vi "Dresden R2R Sputter 03.02.2018 IY24.vi"() -> ()   [LabVIEW 2009] (continued)
                        n5703 = while {
                          i -> [w8756]
                          stop <- w8751 stop-if-true
                          n5704 = Greater?(x=w8756, y=100) -> (0:w8752:bool)
                          n5705 = Wait Until Next ms Multiple(millisecond multiple=u32 300) -> ()  [unwired: 1 out]
                          n5706 = local read "Parameters_auto_set"() -> (w8757:bool)
                          n5707 = case shown="False" w8757 {
                            tunnel: [TRUE FALSE] -> w8753
                            frame #0 {
                            }
                            frame #1 {
                            }
                          }
                          n5708 = Or(x=w8753, y=w8752) -> (x .or. y?=w8751:bool)
                        }
                      }
                      frame #9 {
                        n5709 = local write "Start_roll"(TRUE ("Start_roll")) -> ()
                      }
                      frame #10 {
                        n5710 = while {
                          stop <- w8762 stop-if-true
                          n5711 = local read "Actual Length"() -> (w8766:dbl)
                          n5712 = local read "Region"() -> (w8765:dbl)
                          n5713 = local read "Semi"() -> (w8763:bool)
                          n5714 = Greater Or Equal?(x=w8766, y=w8765) -> (x >= y?=w8764:bool)
                          n5715 = Or(x=w8764, y=w8763) -> (x .or. y?=w8762:bool)
                          n5716 = Wait Until Next ms Multiple(millisecond multiple=u32 300) -> ()  [unwired: 1 out]
                        }
                      }
                      frame #11 {
                        n5717 = local write "Start_full_foil"(FALSE ("Start_full_foil")) -> ()
                      }
                    }
                  }
                }
              }
              frame #1 {
                n5718 = local read "Roll_side_select 2"() -> (w8768:enum32{"Left to Right", "Right to Left"})
                n5719 = case shown="\"Right to Left\"" w8768 {
                  frame #0 {
                    n5720 = stacked-sequence {
                      frame #0 {
                        n5721 = local read "Target_length_left side"() -> (w8772:dbl)
                        n5722 = local read "Max Diameter 2"() -> (w8775:dbl)
                        n5723 = local read "Min Diameter 2"() -> (w8774:dbl)
                        n5724 = local read "Web Speed 2"() -> (w8770:dbl)
                        n5725 = local read "Web_Thickness2"() -> (w8769:dbl)
                        n5726 = local write "Initial Min Diameter"(w8774) -> ()
                        n5727 = local write "Web Speed"(w8770) -> ()
                        n5728 = local write "Max Diameter"(w8775) -> ()
                        n5729 = local write "Roll_side_select"(enum32{"Left to Right", "Right to Left"}."Left to Right" ("Roll_side_select")) -> ()
                        n5730 = local write "Region"(w8772) -> ()
                        n5731 = local write "Web Thickness"(w8769) -> ()
                        n5732 = Wait (ms)(milliseconds to wait=u32 1000) -> ()  [unwired: 1 out]
                      }
                      frame #1 {
                        n5733 = local write "Calculate 2"(TRUE ("Calculate_auto")) -> ()
                      }
                      frame #2 {
                        n5734 = local read "Tension_Value2"() -> (w8778:dbl)
                        n5735 = Wait (ms)(milliseconds to wait=u32 300) -> ()  [unwired: 1 out]
                        n5736 = local write "TC1_set_value"(w8778) -> ()
                      }
                      frame #3 {
                        w8779 = u16 1 items=["1", "2", "3", "4"] ("Target Chamber Sensor")
                        n5737 = local write "Target Chamber Sensor"(w8779) -> ()
                      }
                      frame #4 {
                        n5738 = local write "TC1_set"(TRUE ("TC1_set")) -> ()
                      }
                      frame #5 {
                        n5739 = local write "Parameters_auto_set"(TRUE ("Parameters_auto_set")) -> ()
                      }
                      frame #6 {
                        n5740 = while {
                          i -> [w8787]
                          stop <- w8782 stop-if-true
                          n5741 = Greater?(x=w8787, y=100) -> (0:w8783:bool)
                          n5742 = Wait Until Next ms Multiple(millisecond multiple=u32 300) -> ()  [unwired: 1 out]
                          n5743 = local read "Parameters_auto_set"() -> (w8788:bool)
                          n5744 = case shown="False" w8788 {
                            tunnel: [TRUE FALSE] -> w8784
                            frame #0 {
                            }
                            frame #1 {
                            }
                          }
                          n5745 = Or(x=w8784, y=w8783) -> (x .or. y?=w8782:bool)
                        }
                      }
                      frame #7 {
                        n5746 = local write "Start_roll"(TRUE ("Start_roll")) -> ()
                      }
                      frame #8 {
                        n5747 = while {
                          stop <- w8793 stop-if-true
                          n5748 = local read "Actual Length"() -> (w8797:dbl)
                          n5749 = local read "Region"() -> (w8796:dbl)
                          n5750 = local read "Semi"() -> (w8794:bool)
                          n5751 = Greater Or Equal?(x=w8797, y=w8796) -> (x >= y?=w8795:bool)
                          n5752 = Or(x=w8795, y=w8794) -> (x .or. y?=w8793:bool)
                          n5753 = Wait Until Next ms Multiple(millisecond multiple=u32 300) -> ()  [unwired: 1 out]
                        }
                      }
                      frame #9 {
                        n5754 = local write "Start_full_foil"(FALSE ("Start_full_foil")) -> ()
                      }
                    }
                  }
                  frame #1 {
                    n5755 = stacked-sequence {
                      frame #0 {
                        n5756 = local read "Target_length_right side"() -> (w8803:dbl)
                        n5757 = local read "Web_Thickness2"() -> (w8799:dbl)
                        n5758 = local read "Max Diameter 2"() -> (w8804:dbl)
                        n5759 = local read "Web Speed 2"() -> (w8800:dbl)
                        n5760 = local write "Web Speed"(w8800) -> ()
                        n5761 = local write "Max Diameter"(w8804) -> ()
                        n5762 = local write "Roll_side_select"(enum32{"Left to Right", "Right to Left"}."Right to Left" ("Roll_side_select")) -> ()
                        n5763 = local write "Web Thickness"(w8799) -> ()
                        n5764 = local write "Region"(w8803) -> ()
                        n5765 = Wait (ms)(milliseconds to wait=u32 1000) -> ()  [unwired: 1 out]
                      }
                      frame #1 {
                        n5766 = local write "Calculate 3"(TRUE ("Calculate_auto")) -> ()
                      }
                      frame #2 {
                        n5767 = local read "Change_Max Diameter"() -> (w8807:dbl)
                        n5768 = Wait (ms)(milliseconds to wait=u32 300) -> ()  [unwired: 1 out]
                        n5769 = local write "Initial Min Diameter"(w8807) -> ()
                      }
                      frame #3 {
                        n5770 = local write "Calculate 2"(TRUE ("Calculate_auto")) -> ()
                      }
                      frame #4 {
                        w8809 = u16 1 items=["1", "2", "3", "4"] ("Target Chamber Sensor")
                        n5771 = local write "Target Chamber Sensor"(w8809) -> ()
                      }
                      frame #5 {
                        n5772 = local read "Tension_Value2"() -> (w8811:dbl)
                        n5773 = Wait (ms)(milliseconds to wait=u32 300) -> ()  [unwired: 1 out]
                        n5774 = local write "TC2_set_value"(w8811) -> ()
                      }
                      frame #6 {
                        n5775 = local write "TC2_set"(TRUE ("TC1_set")) -> ()
                      }
                      frame #7 {
                        n5776 = local write "Parameters_auto_set"(TRUE ("Parameters_auto_set")) -> ()
                      }
                      frame #8 {
                        n5777 = while {
                          i -> [w8819]
                          stop <- w8814 stop-if-true
                          n5778 = Greater?(x=w8819, y=100) -> (0:w8815:bool)
                          n5779 = Wait Until Next ms Multiple(millisecond multiple=u32 300) -> ()  [unwired: 1 out]
                          n5780 = local read "Parameters_auto_set"() -> (w8820:bool)
                          n5781 = case shown="False" w8820 {
                            tunnel: [TRUE FALSE] -> w8816
                            frame #0 {
                            }
                            frame #1 {
                            }
                          }
                          n5782 = Or(x=w8816, y=w8815) -> (x .or. y?=w8814:bool)
                        }
                      }
                      frame #9 {
                        n5783 = local write "Start_roll"(TRUE ("Start_roll")) -> ()
                      }
                      frame #10 {
                        n5784 = while {
                          stop <- w8825 stop-if-true
                          n5785 = local read "Actual Length"() -> (w8829:dbl)
                          n5786 = local read "Region"() -> (w8828:dbl)
                          n5787 = local read "Semi"() -> (w8826:bool)
                          n5788 = Greater Or Equal?(x=w8829, y=w8828) -> (x >= y?=w8827:bool)
                          n5789 = Or(x=w8827, y=w8826) -> (x .or. y?=w8825:bool)
                          n5790 = Wait Until Next ms Multiple(millisecond multiple=u32 300) -> ()  [unwired: 1 out]
                        }
                      }
                      frame #11 {
                        n5791 = local write "Start_full_foil"(FALSE ("Start_full_foil")) -> ()
                      }
                    }
                  }
                }
              }
              frame #2 {
                n5792 = local read "Roll_side_select 2"() -> (w8831:enum32{"Left to Right", "Right to Left"})
                n5793 = case shown="\"Left to Right\", Default" w8831 {
                  frame #0 {
                    n5794 = stacked-sequence {
                      frame #0 {
                        n5795 = local read "Target_length_left side"() -> (w8835:dbl)
                        n5796 = local read "Max Diameter 2"() -> (w8838:dbl)
                        n5797 = local read "Min Diameter 2"() -> (w8837:dbl)
                        n5798 = local read "Web_Thickness2"() -> (w8832:dbl)
                        n5799 = local read "Web Speed 2"() -> (w8833:dbl)
                        n5800 = local write "Initial Min Diameter"(w8837) -> ()
                        n5801 = local write "Web Speed"(w8833) -> ()
                        n5802 = local write "Max Diameter"(w8838) -> ()
                        n5803 = local write "Roll_side_select"(enum32{"Left to Right", "Right to Left"}."Left to Right" ("Roll_side_select")) -> ()
                        n5804 = local write "Web Thickness"(w8832) -> ()
                        n5805 = local write "Region"(w8835) -> ()
                        n5806 = Wait (ms)(milliseconds to wait=u32 1000) -> ()  [unwired: 1 out]
                      }
                      frame #1 {
                        n5807 = local write "Calculate 2"(TRUE ("Calculate_auto")) -> ()
                      }
                      frame #2 {
                        n5808 = local read "Tension_Value2"() -> (w8841:dbl)
                        n5809 = Wait (ms)(milliseconds to wait=u32 300) -> ()  [unwired: 1 out]
                        n5810 = local write "TC1_set_value"(w8841) -> ()
                      }
                      frame #3 {
                        w8842 = u16 2 items=["1", "2", "3", "4"] ("Target Chamber Sensor")
                        n5811 = local write "Target Chamber Sensor"(w8842) -> ()
                      }
                      frame #4 {
                        n5812 = local write "TC1_set"(TRUE ("TC1_set")) -> ()
                      }
                      frame #5 {
                        n5813 = local write "Parameters_auto_set"(TRUE ("Parameters_auto_set")) -> ()
                      }
                      frame #6 {
                        n5814 = while {
                          i -> [w8850]
                          stop <- w8845 stop-if-true
                          n5815 = Greater?(x=w8850, y=100) -> (0:w8846:bool)
                          n5816 = Wait Until Next ms Multiple(millisecond multiple=u32 300) -> ()  [unwired: 1 out]
                          n5817 = local read "Parameters_auto_set"() -> (w8851:bool)
                          n5818 = case shown="False" w8851 {
                            tunnel: [TRUE FALSE] -> w8847
                            frame #0 {
                            }
                            frame #1 {
                            }
                          }
                          n5819 = Or(x=w8847, y=w8846) -> (x .or. y?=w8845:bool)
                        }
                      }
                      frame #7 {
                        n5820 = local write "Start_roll"(TRUE ("Start_roll")) -> ()
                      }
                      frame #8 {
                        n5821 = while {
                          stop <- w8856 stop-if-true
                          n5822 = local read "Actual Length"() -> (w8860:dbl)
                          n5823 = local read "Region"() -> (w8859:dbl)
                          n5824 = local read "Semi"() -> (w8857:bool)
                          n5825 = Greater Or Equal?(x=w8860, y=w8859) -> (x >= y?=w8858:bool)
                          n5826 = Or(x=w8858, y=w8857) -> (x .or. y?=w8856:bool)
                          n5827 = Wait Until Next ms Multiple(millisecond multiple=u32 300) -> ()  [unwired: 1 out]
                        }
                      }
                      frame #9 {
                        n5828 = local write "Start_full_foil"(FALSE ("Start_full_foil")) -> ()
                      }
                    }
                  }
                  frame #1 {
                    n5829 = stacked-sequence {
                      frame #0 {
                        n5830 = local read "Target_length_right side"() -> (w8866:dbl)
                        n5831 = local read "Max Diameter 2"() -> (w8867:dbl)
                        n5832 = local read "Web_Thickness2"() -> (w8862:dbl)
                        n5833 = local read "Web Speed 2"() -> (w8863:dbl)
                        n5834 = local write "Web Speed"(w8863) -> ()
                        n5835 = local write "Max Diameter"(w8867) -> ()
                        n5836 = local write "Roll_side_select"(enum32{"Left to Right", "Right to Left"}."Right to Left" ("Roll_side_select")) -> ()
                        n5837 = local write "Web Thickness"(w8862) -> ()
                        n5838 = local write "Region"(w8866) -> ()
                        n5839 = Wait (ms)(milliseconds to wait=u32 1000) -> ()  [unwired: 1 out]
                      }
                      frame #1 {
                        n5840 = local write "Calculate 3"(TRUE ("Calculate_auto")) -> ()
                      }
                      frame #2 {
                        n5841 = local read "Change_Max Diameter"() -> (w8870:dbl)
                        n5842 = Wait (ms)(milliseconds to wait=u32 300) -> ()  [unwired: 1 out]
                        n5843 = local write "Initial Min Diameter"(w8870) -> ()
                      }
                      frame #3 {
                        n5844 = local write "Calculate 2"(TRUE ("Calculate_auto")) -> ()
                      }
                      frame #4 {
                        w8872 = u16 2 items=["1", "2", "3", "4"] ("Target Chamber Sensor")
                        n5845 = local write "Target Chamber Sensor"(w8872) -> ()
                      }
                      frame #5 {
                        n5846 = local read "Tension_Value2"() -> (w8874:dbl)
                        n5847 = Wait (ms)(milliseconds to wait=u32 300) -> ()  [unwired: 1 out]
                        n5848 = local write "TC2_set_value"(w8874) -> ()
                      }
                      frame #6 {
                        n5849 = local write "TC2_set"(TRUE ("TC1_set")) -> ()
                      }
                      frame #7 {
                        n5850 = local write "Parameters_auto_set"(TRUE ("Parameters_auto_set")) -> ()
                      }
                      frame #8 {
                        n5851 = while {
                          i -> [w8882]
                          stop <- w8877 stop-if-true
                          n5852 = Greater?(x=w8882, y=100) -> (0:w8878:bool)
                          n5853 = Wait Until Next ms Multiple(millisecond multiple=u32 300) -> ()  [unwired: 1 out]
                          n5854 = local read "Parameters_auto_set"() -> (w8883:bool)
                          n5855 = case shown="False" w8883 {
                            tunnel: [TRUE FALSE] -> w8879
                            frame #0 {
                            }
                            frame #1 {
                            }
                          }
                          n5856 = Or(x=w8879, y=w8878) -> (x .or. y?=w8877:bool)
                        }
                      }
                      frame #9 {
                        n5857 = local write "Start_roll"(TRUE ("Start_roll")) -> ()
                      }
                      frame #10 {
                        n5858 = while {
                          stop <- w8888 stop-if-true
                          n5859 = local read "Actual Length"() -> (w8892:dbl)
                          n5860 = local read "Region"() -> (w8891:dbl)
                          n5861 = local read "Semi"() -> (w8889:bool)
                          n5862 = Greater Or Equal?(x=w8892, y=w8891) -> (x >= y?=w8890:bool)
                          n5863 = Or(x=w8890, y=w8889) -> (x .or. y?=w8888:bool)
                          n5864 = Wait Until Next ms Multiple(millisecond multiple=u32 300) -> ()  [unwired: 1 out]
                        }
                      }
                      frame #11 {
                        n5865 = local write "Start_full_foil"(FALSE ("Start_full_foil")) -> ()
                      }
                    }
                  }
                }
              }
              frame #3 {
                n5866 = local read "Roll_side_select 2"() -> (w8894:enum32{"Left to Right", "Right to Left"})
                n5867 = case shown="\"Right to Left\"" w8894 {
                  frame #0 {
                    n5868 = stacked-sequence {
                      frame #0 {
                        n5869 = local read "Target_length_left side"() -> (w8898:dbl)
                        n5870 = local read "Web_Thickness2"() -> (w8895:dbl)
                        n5871 = local read "Max Diameter 2"() -> (w8901:dbl)
                        n5872 = local read "Min Diameter 2"() -> (w8900:dbl)
                        n5873 = local read "Web Speed 2"() -> (w8896:dbl)
                        n5874 = local write "Web Thickness"(w8895) -> ()
                        n5875 = local write "Initial Min Diameter"(w8900) -> ()
                        n5876 = local write "Web Speed"(w8896) -> ()
                        n5877 = local write "Max Diameter"(w8901) -> ()
                        n5878 = local write "Roll_side_select"(enum32{"Left to Right", "Right to Left"}."Left to Right" ("Roll_side_select")) -> ()
                        n5879 = local write "Region"(w8898) -> ()
                        n5880 = Wait (ms)(milliseconds to wait=u32 1000) -> ()  [unwired: 1 out]
                      }
                      frame #1 {
                        n5881 = local write "Calculate 2"(TRUE ("Calculate_auto")) -> ()
                      }
                      frame #2 {
                        n5882 = local read "Tension_Value2"() -> (w8904:dbl)
                        n5883 = Wait (ms)(milliseconds to wait=u32 300) -> ()  [unwired: 1 out]
                        n5884 = local write "TC1_set_value"(w8904) -> ()
                      }
                      frame #3 {
                        w8905 = u16 3 items=["1", "2", "3", "4"] ("Target Chamber Sensor")
                        n5885 = local write "Target Chamber Sensor"(w8905) -> ()
                      }
                      frame #4 {
                        n5886 = local write "TC1_set"(TRUE ("TC1_set")) -> ()
                      }
                      frame #5 {
                        n5887 = local write "Parameters_auto_set"(TRUE ("Parameters_auto_set")) -> ()
                      }
                      frame #6 {
                        n5888 = while {
                          i -> [w8913]
                          stop <- w8908 stop-if-true
                          n5889 = Greater?(x=w8913, y=100) -> (0:w8909:bool)
                          n5890 = Wait Until Next ms Multiple(millisecond multiple=u32 300) -> ()  [unwired: 1 out]
                          n5891 = local read "Parameters_auto_set"() -> (w8914:bool)
                          n5892 = case shown="False" w8914 {
                            tunnel: [TRUE FALSE] -> w8910
                            frame #0 {
                            }
                            frame #1 {
                            }
                          }
                          n5893 = Or(x=w8910, y=w8909) -> (x .or. y?=w8908:bool)
                        }
                      }
                      frame #7 {
                        n5894 = local write "Start_roll"(TRUE ("Start_roll")) -> ()
                      }
                      frame #8 {
                        n5895 = while {
                          stop <- w8919 stop-if-true
                          n5896 = local read "Actual Length"() -> (w8923:dbl)
                          n5897 = local read "Region"() -> (w8922:dbl)
                          n5898 = local read "Semi"() -> (w8920:bool)
                          n5899 = Greater Or Equal?(x=w8923, y=w8922) -> (x >= y?=w8921:bool)
                          n5900 = Or(x=w8921, y=w8920) -> (x .or. y?=w8919:bool)
                          n5901 = Wait Until Next ms Multiple(millisecond multiple=u32 300) -> ()  [unwired: 1 out]
                        }
                      }
                      frame #9 {
                        n5902 = local write "Start_full_foil"(FALSE ("Start_full_foil")) -> ()
                      }
                    }
                  }
                  frame #1 {
                    n5903 = stacked-sequence {
                      frame #0 {
                        n5904 = local read "Target_length_right side"() -> (w8929:dbl)
                        n5905 = local read "Web_Thickness2"() -> (w8925:dbl)
                        n5906 = local read "Max Diameter 2"() -> (w8930:dbl)
                        n5907 = local read "Web Speed 2"() -> (w8926:dbl)
                        n5908 = local write "Web Thickness"(w8925) -> ()
                        n5909 = local write "Web Speed"(w8926) -> ()
                        n5910 = local write "Max Diameter"(w8930) -> ()
                        n5911 = local write "Roll_side_select"(enum32{"Left to Right", "Right to Left"}."Right to Left" ("Roll_side_select")) -> ()
                        n5912 = local write "Region"(w8929) -> ()
                        n5913 = Wait (ms)(milliseconds to wait=u32 1000) -> ()  [unwired: 1 out]
                      }
                      frame #1 {
                        n5914 = local write "Calculate 3"(TRUE ("Calculate_auto")) -> ()
                      }
                      frame #2 {
                        n5915 = local read "Change_Max Diameter"() -> (w8933:dbl)
                        n5916 = Wait (ms)(milliseconds to wait=u32 300) -> ()  [unwired: 1 out]
                        n5917 = local write "Initial Min Diameter"(w8933) -> ()
                      }
                      frame #3 {
                        n5918 = local write "Calculate 2"(TRUE ("Calculate_auto")) -> ()
                      }
                      frame #4 {
                        w8935 = u16 3 items=["1", "2", "3", "4"] ("Target Chamber Sensor")
                        n5919 = local write "Target Chamber Sensor"(w8935) -> ()
                      }
                      frame #5 {
                        n5920 = local read "Tension_Value2"() -> (w8937:dbl)
                        n5921 = Wait (ms)(milliseconds to wait=u32 300) -> ()  [unwired: 1 out]
                        n5922 = local write "TC2_set_value"(w8937) -> ()
                      }
                      frame #6 {
                        n5923 = local write "TC2_set"(TRUE ("TC1_set")) -> ()
                      }
                      frame #7 {
                        n5924 = local write "Parameters_auto_set"(TRUE ("Parameters_auto_set")) -> ()
                      }
                      frame #8 {
                        n5925 = while {
                          i -> [w8945]
                          stop <- w8940 stop-if-true
                          n5926 = Greater?(x=w8945, y=100) -> (0:w8941:bool)
                          n5927 = Wait Until Next ms Multiple(millisecond multiple=u32 300) -> ()  [unwired: 1 out]
                          n5928 = local read "Parameters_auto_set"() -> (w8946:bool)
                          n5929 = case shown="False" w8946 {
                            tunnel: [TRUE FALSE] -> w8942
                            frame #0 {
                            }
                            frame #1 {
                            }
                          }
                          n5930 = Or(x=w8942, y=w8941) -> (x .or. y?=w8940:bool)
                        }
                      }
                      frame #9 {
                        n5931 = local write "Start_roll"(TRUE ("Start_roll")) -> ()
                      }
                      frame #10 {
                        n5932 = while {
                          stop <- w8951 stop-if-true
                          n5933 = local read "Actual Length"() -> (w8955:dbl)
                          n5934 = local read "Region"() -> (w8954:dbl)
                          n5935 = local read "Semi"() -> (w8952:bool)
                          n5936 = Greater Or Equal?(x=w8955, y=w8954) -> (x >= y?=w8953:bool)
                          n5937 = Or(x=w8953, y=w8952) -> (x .or. y?=w8951:bool)
                          n5938 = Wait Until Next ms Multiple(millisecond multiple=u32 300) -> ()  [unwired: 1 out]
                        }
                      }
                      frame #11 {
                        n5939 = local write "Start_full_foil"(FALSE ("Start_full_foil")) -> ()
                      }
                    }
                  }
                }
              }
            }
          }
        }
      }
    }
    n5940 = local read "Roll_Selection"() -> (w8544:enum32{"Full_foil", "Specified Length of Foil"})
    n5941 = case shown="\"Full_foil\", Default" w8544 {
      frame #0 {
        n5942 = local write "Roll_calculation_tab"(T15."Specified Length of Foil " ("Roll_calculation_tab")) -> ()
      }
      frame #1 {
        n5943 = local read "Roll_side_select 2"() -> (w8547:enum32{"Left to Right", "Right to Left"})
        n5944 = local write "Roll_calculation_tab"(T15."Specified Length of Foil " ("Roll_calculation_tab")) -> ()
        n5945 = case shown="\"Left to Right\", Default" w8547 {
          frame #0 {
            n5946 = local write "Specified Control"(T16."Left to Right                " ("Specified Control")) -> ()
          }
          frame #1 {
            n5947 = local write "Specified Control"(T16."Right to Left                  " ("Specified Control")) -> ()
          }
        }
      }
    }
  }
  n5948 = while {
    stop <- FALSE stop-if-true
    n5949 = Wait Until Next ms Multiple(millisecond multiple=u32 100) -> ()  [unwired: 1 out]
    n5950 = case shown="True" "Calculate 3" {
      frame #0 {
      }
      frame #1 {
        n5951 = stacked-sequence {
          frame #0 {
            n5952 = local write "Calculate 3"(FALSE ("Calculate 2")) -> ()
            n5953 = Wait (ms)(milliseconds to wait=u32 100) -> ()  [unwired: 1 out]
          }
          frame #1 {
            w8969 = 0.0 ("Region")
            n5954 = local read "Max Diameter"() -> (w8970:dbl)
            n5955 = local write "Change_Max Diameter"(w8970) -> ()
            n5956 = local write "Actual Diameter"(w8970) -> ()
            n5957 = Wait (ms)(milliseconds to wait=u32 1000) -> ()  [unwired: 1 out]
            n5958 = local write "Region 3"(w8969) -> ()
            n5959 = local write "Lap 3"(w8969) -> ()
          }
          frame #2 {
            n5960 = while {
              stop <- w8973 stop-if-true
              n5961 = local read "Change_Max Diameter"() -> (w8984:dbl)
              n5962 = local read "Lap 3"() -> (w8981:dbl)
              n5963 = local read "Web Thickness"() -> (w8983:dbl)
              n5964 = Increment(x=w8981) -> (x+1=w8972:dbl)
              n5965 = local read "Change_Max Diameter"() -> (w8976:dbl)
              n5966 = local write "Lap 3"(w8972) -> ()
              n5967 = Multiply(x=w8983, y=0.002) -> (x*y=w8986:dbl)
              n5968 = Subtract(x=w8984, y=w8986) -> (x-y=w8982:dbl)
              n5969 = local write "Change_Max Diameter"(w8982) -> ()
              n5970 = Multiply(x=w8976, y=3.14) -> (x*y=w8979:dbl)
              n5971 = local read "Region 3"() -> (w8975:dbl)
              n5972 = Divide(x=w8979, y=1000.0) -> (x/y=w8977:dbl)
              n5973 = Add(x=w8977, y=w8975) -> (x+y=w8971:dbl)
              n5974 = local read "Total length"() -> (w8974:dbl)
              n5975 = local write "Region 3"(w8971) -> ()
              n5976 = Greater Or Equal?(x=w8971, y=w8974) -> (x >= y?=w8973:bool)
              n5977 = Wait Until Next ms Multiple(millisecond multiple=u32 10) -> ()  [unwired: 1 out]
            }
          }
          frame #3 {
            n5978 = local read "Change_Max Diameter"() -> (w8990:dbl)
            n5979 = local read "Max Diameter"() -> (w8989:dbl)
            n5980 = local read "Web Speed"() -> (w8991:dbl)
            n5981 = Divide(x=w8990, y=2.0) -> (x/y=w9008:dbl)
            n5982 = Multiply(x=3.141592653589793, y=2.0) -> (x*y=w8997:dbl)
            n5983 = Multiply(x=w9008, y=w8997) -> (x*y=w9005:dbl)
            n5984 = Divide(x=w8989, y=2.0) -> (x/y=w9001:dbl)
            n5985 = Multiply(x=3.141592653589793, y=2.0) -> (x*y=w8994:dbl)
            n5986 = Multiply(x=w9001, y=w8994) -> (x*y=w9004:dbl)
            n5987 = Divide(x=w8991, y=w9005) -> (x/y=w9007:dbl)
            n5988 = Divide(x=w8991, y=w9004) -> (x/y=w9002:dbl)
            n5989 = Multiply(x=w9007, y=10.0) -> (x*y=w8993:dbl)
            n5990 = Multiply(x=w9002, y=10.0) -> (x*y=w8992:dbl)
            n5991 = local write "Max Circular Speed"(w8993) -> ()
            n5992 = local write "Min Circular Speed"(w8992) -> ()
            n5993 = Wait (ms)(milliseconds to wait=u32 200) -> ()  [unwired: 1 out]
          }
          frame #4 {
            n5994 = local read "Max Circular Speed"() -> (w9012:dbl)
            n5995 = Divide(x=w9012, y=2.0) -> (x/y=w9011:dbl)
            n5996 = Wait (ms)(milliseconds to wait=u32 100) -> ()  [unwired: 1 out]
            n5997 = local write "Output voltage value"(w9011) -> ()
          }
          frame #5 {
            # "reduction ratio"
            n5998 = local read "Speed-voltage constant"() -> (w9015:dbl)
            n5999 = local read "Max Circular Speed"() -> (w9019:dbl)
            n6000 = local read "Min Circular Speed"() -> (w9016:dbl)
            n6001 = Multiply(x=w9015, y=50.0) -> (x*y=w9023:dbl)
            n6002 = Multiply(x=w9019, y=w9023) -> (x*y=w9022:dbl)
            n6003 = Multiply(x=w9023, y=w9016) -> (x*y=w9021:dbl)
            n6004 = local read "Lap 3"() -> (w9020:dbl)
            n6005 = Subtract(x=w9022, y=w9021) -> (x-y=w9017:dbl)
            n6006 = Divide(x=w9017, y=w9020) -> (x/y=w9018:dbl)
            n6007 = local write "Voltage difference value"(w9017) -> ()
            n6008 = local write "Set voltage value"(w9018) -> ()
            n6009 = Wait (ms)(milliseconds to wait=u32 100) -> ()  [unwired: 1 out]
          }
          frame #6 {
            n6010 = local read "Region 3"() -> (w9026:dbl)
            n6011 = local write "Region"(w9026) -> ()
            n6012 = Wait (ms)(milliseconds to wait=u32 100) -> ()  [unwired: 1 out]
          }
        }
      }
    }
    n6013 = case shown="True" "Calculate 2" {
      frame #0 {
      }
      frame #1 {
        n6014 = stacked-sequence {
          frame #0 {
            n6015 = local write "Calculate 2"(FALSE ("Calculate 2")) -> ()
            n6016 = Wait (ms)(milliseconds to wait=u32 100) -> ()  [unwired: 1 out]
          }
          frame #1 {
            w9029 = 0.0 ("Lap")
            n6017 = local read "Change_Min Diameter"() -> (w9030:dbl)
            n6018 = local read "Initial Min Diameter"() -> (w9032:dbl)
            n6019 = local write "Actual Diameter"(w9030) -> ()
            n6020 = local write "Change_Min Diameter"(w9032) -> ()
            n6021 = Wait (ms)(milliseconds to wait=u32 1000) -> ()  [unwired: 1 out]
            n6022 = local write "Region 2"(w9029) -> ()
            n6023 = local write "Lap 2"(w9029) -> ()
          }
          frame #2 {
            n6024 = while {
              stop <- w9043 stop-if-true
              n6025 = local read "Change_Min Diameter"() -> (w9048:dbl)
              n6026 = local read "Web Thickness"() -> (w9035:dbl)
              n6027 = Wait Until Next ms Multiple(millisecond multiple=u32 10) -> ()  [unwired: 1 out]
              n6028 = local read "Lap 2"() -> (w9045:dbl)
              n6029 = Multiply(x=w9035, y=0.002) -> (x*y=w9047:dbl)
              n6030 = Add(x=w9048, y=w9047) -> (x+y=w9046:dbl)
              n6031 = Increment(x=w9045) -> (x+1=w9034:dbl)
              n6032 = local write "Change_Min Diameter"(w9046) -> ()
              n6033 = local write "Lap 2"(w9034) -> ()
              n6034 = local read "Change_Min Diameter"() -> (w9040:dbl)
              n6035 = local read "Total length"() -> (w9036:dbl)
              n6036 = Multiply(x=w9040, y=3.141592653589793) -> (x*y=w9041:dbl)
              n6037 = local read "Region 2"() -> (w9038:dbl)
              n6038 = Divide(x=w9041, y=1000.0) -> (x/y=w9042:dbl)
              n6039 = Add(x=w9042, y=w9038) -> (x+y=w9033:dbl)
              n6040 = Greater Or Equal?(x=w9033, y=w9036) -> (x >= y?=w9043:bool)
              n6041 = local write "Region 2"(w9033) -> ()
            }
          }
          frame #3 {
            n6042 = local read "Initial Min Diameter"() -> (w9051:dbl)
            n6043 = local read "Change_Min Diameter"() -> (w9055:dbl)
            n6044 = local read "Web Speed"() -> (w9052:dbl)
            n6045 = Divide(x=w9051, y=2.0) -> (x/y=w9069:dbl)
            n6046 = Multiply(x=3.141592653589793, y=2.0) -> (x*y=w9058:dbl)
            n6047 = Multiply(x=w9069, y=w9058) -> (x*y=w9066:dbl)
            n6048 = Divide(x=w9055, y=2.0) -> (x/y=w9062:dbl)
            n6049 = Multiply(x=3.141592653589793, y=2.0) -> (x*y=w9056:dbl)
            n6050 = Multiply(x=w9062, y=w9056) -> (x*y=w9065:dbl)
            n6051 = Divide(x=w9052, y=w9066) -> (x/y=w9068:dbl)
            n6052 = Divide(x=w9052, y=w9065) -> (x/y=w9063:dbl)
            n6053 = Multiply(x=w9068, y=10.0) -> (x*y=w9054:dbl)
            n6054 = Multiply(x=w9063, y=10.0) -> (x*y=w9053:dbl)
            n6055 = local write "Max Circular Speed"(w9054) -> ()
            n6056 = local write "Min Circular Speed"(w9053) -> ()
            n6057 = Wait (ms)(milliseconds to wait=u32 100) -> ()  [unwired: 1 out]
          }
          frame #4 {
            n6058 = local read "Max Circular Speed"() -> (w9074:dbl)
            n6059 = Divide(x=w9074, y=2.0) -> (x/y=w9073:dbl)
            n6060 = Wait (ms)(milliseconds to wait=u32 100) -> ()  [unwired: 1 out]
            n6061 = local write "Output voltage value"(w9073) -> ()
          }
          frame #5 {
            # "reduction ratio"
            n6062 = local read "Speed-voltage constant"() -> (w9077:dbl)
            n6063 = local read "Max Circular Speed"() -> (w9081:dbl)
            n6064 = local read "Min Circular Speed"() -> (w9078:dbl)
            n6065 = Multiply(x=w9077, y=50.0) -> (x*y=w9085:dbl)
            n6066 = Multiply(x=w9081, y=w9085) -> (x*y=w9084:dbl)
            n6067 = Multiply(x=w9085, y=w9078) -> (x*y=w9083:dbl)
            n6068 = Subtract(x=w9084, y=w9083) -> (x-y=w9079:dbl)
            n6069 = local read "Lap 2"() -> (w9082:dbl)
            n6070 = Divide(x=w9079, y=w9082) -> (x/y=w9080:dbl)
            n6071 = local write "Voltage difference value"(w9079) -> ()
            n6072 = local write "Set voltage value"(w9080) -> ()
            n6073 = Wait (ms)(milliseconds to wait=u32 100) -> ()  [unwired: 1 out]
          }
          frame #6 {
            n6074 = local read "Region 2"() -> (w9088:dbl)
            n6075 = local write "Region"(w9088) -> ()
            n6076 = Wait (ms)(milliseconds to wait=u32 100) -> ()  [unwired: 1 out]
          }
        }
      }
    }
    n6077 = case shown="True" "Calculate_auto" {
      frame #0 {
      }
      frame #1 {
        n6078 = stacked-sequence {
          frame #0 {
            w9212 = 0.0 ("Region")
            n6079 = local read "Min Diameter"() -> (w9211:dbl)
            n6080 = Wait (ms)(milliseconds to wait=u32 1000) -> ()  [unwired: 1 out]
            n6081 = local write "Diameter"(w9211) -> ()
            n6082 = local write "Actual Diameter"(w9211) -> ()
            n6083 = local write "Region1"(w9212) -> ()
            n6084 = local write "Lap"(w9212) -> ()
          }
          frame #1 {
            n6085 = while {
              stop <- w9221 stop-if-true
              n6086 = local read "Web Thickness"() -> (w9218:dbl)
              n6087 = local read "Diameter"() -> (w9217:dbl)
              n6088 = Wait Until Next ms Multiple(millisecond multiple=u32 10) -> ()  [unwired: 1 out]
              n6089 = Multiply(x=w9218, y=0.002) -> (x*y=w9229:dbl)
              n6090 = local read "Lap"() -> (w9219:dbl)
              n6091 = Add(x=w9217, y=w9229) -> (x+y=w9224:dbl)
              n6092 = Increment(x=w9219) -> (x+1=w9216:dbl)
              n6093 = local write "Diameter"(w9224) -> ()
              n6094 = local write "Lap"(w9216) -> ()
              n6095 = local read "Max Diameter"() -> (w9223:dbl)
              n6096 = local read "Diameter"() -> (w9222:dbl)
              n6097 = Greater Or Equal?(x=w9222, y=w9223) -> (x >= y?=w9221:bool)
              n6098 = Multiply(x=w9222, y=3.141592653589793) -> (x*y=w9225:dbl)
              n6099 = Divide(x=w9225, y=1000.0) -> (x/y=w9227:dbl)
              n6100 = local read "Region1"() -> (w9228:dbl)
              n6101 = Add(x=w9227, y=w9228) -> (x+y=w9215:dbl)
              n6102 = local write "Region1"(w9215) -> ()
            }
          }
          frame #2 {
            w9239 = 10.0 ("y")
            n6103 = local read "Max Diameter"() -> (w9235:dbl)
            n6104 = local read "Min Diameter"() -> (w9242:dbl)
            n6105 = local read "Web Speed"() -> (w9234:dbl)
            n6106 = Divide(x=w9235, y=2.0) -> (x/y=w9245:dbl)
            n6107 = Divide(x=w9242, y=2.0) -> (x/y=w9246:dbl)
            n6108 = Multiply(x=w9245, y=6.28) -> (x*y=w9244:dbl)
            n6109 = Multiply(x=w9246, y=6.28) -> (x*y=w9247:dbl)
            n6110 = Divide(x=w9234, y=w9244) -> (x/y=w9237:dbl)
            n6111 = Divide(x=w9234, y=w9247) -> (x/y=w9238:dbl)
            n6112 = Multiply(x=w9239, y=w9238) -> (x*y=w9232:dbl)
            n6113 = Multiply(x=w9237, y=w9239) -> (x*y=w9233:dbl)
            n6114 = Wait (ms)(milliseconds to wait=u32 100) -> ()  [unwired: 1 out]
            n6115 = local write "Min Circular Speed"(w9233) -> ()
            n6116 = local write "Max Circular Speed"(w9232) -> ()
          }
          frame #3 {
            n6117 = disable-structure shown="Disabled" {
              frame #0 {
                n6118 = local read "Max Circular Speed"() -> (w9250:dbl)
                n6119 = Divide(x=w9250, y=2.0) -> (x/y=w9249:dbl)
                n6120 = local write "Output voltage value"(w9249) -> ()
              }
              frame #1 {
              }
            }
            n6121 = Wait (ms)(milliseconds to wait=u32 100) -> ()  [unwired: 1 out]
          }
          frame #4 {
            n6122 = local read "Speed-voltage constant"() -> (w9255:dbl)
            n6123 = local read "Max Circular Speed"() -> (w9259:dbl)
            n6124 = local read "Min Circular Speed"() -> (w9260:dbl)
            n6125 = Multiply(x=w9255, y=50.0) -> (x*y=w9262:dbl)
            n6126 = Multiply(x=w9259, y=w9262) -> (x*y=w9256:dbl)
            n6127 = Multiply(x=w9262, y=w9260) -> (x*y=w9257:dbl)
            n6128 = Wait (ms)(milliseconds to wait=u32 100) -> ()  [unwired: 1 out]
            n6129 = local read "Lap"() -> (w9258:dbl)
            n6130 = Subtract(x=w9256, y=w9257) -> (x-y=w9253:dbl)
            n6131 = Divide(x=w9253, y=w9258) -> (x/y=w9254:dbl)
            n6132 = local write "Voltage difference value"(w9253) -> ()
            n6133 = local write "Set voltage value"(w9254) -> ()
          }
          frame #5 {
            n6134 = local read "Region1"() -> (w9264:dbl)
            n6135 = Wait (ms)(milliseconds to wait=u32 100) -> ()  [unwired: 1 out]
            n6136 = local write "Region"(w9264) -> ()
          }
          frame #6 {
            n6137 = local write "Calculate_auto"(FALSE ("Calculate_auto")) -> ()
            n6138 = Wait (ms)(milliseconds to wait=u32 100) -> ()  [unwired: 1 out]
          }
        }
      }
    }
    n6139 = case shown="True" "Test_stop" {
      frame #0 {
      }
      frame #1 {
        n6140 = local write "Ch2_SRV_counterclockwise_direction_do"(FALSE ("Ch2_SRV1_direction_do")) -> ()
        n6141 = local write "Ch1_SRV_counterclockwise_direction_do"(FALSE ("Ch2_SRV1_direction_do")) -> ()
        n6142 = local write "Start_roll"(FALSE ("Test_start")) -> ()
        n6143 = local write "Ch2_SRV_start_stop_do"(FALSE ("Ch2_SRV1_start_stop_do")) -> ()
        n6144 = local write "Ch3_SRV_start_stop_do"(FALSE ("Ch2_SRV1_start_stop_do")) -> ()
        n6145 = local write "Ch1_SRV_start_stop_do"(FALSE ("Ch2_SRV1_start_stop_do")) -> ()
        n6146 = Wait (ms)(milliseconds to wait=u32 10) -> ()  [unwired: 1 out]
        n6147 = local write "Ch3_SRV_counterclockwise_direction_do"(FALSE ("Ch2_SRV1_direction_do")) -> ()
        n6148 = local write "Ch4_SRV_counterclockwise_direction_do"(FALSE ("Ch2_SRV1_direction_do")) -> ()
        n6149 = local write "Ch4_SRV_start_stop_do"(FALSE ("Ch2_SRV1_start_stop_do")) -> ()
        n6150 = local write "Test_stop"(FALSE ("Test_stop")) -> ()
        n6151 = local write "Tension_controllers_start/stop_do"(FALSE ("Tension_controllers_start/stop_do")) -> ()
        n6152 = local write "Start_full_foil"(FALSE ("Start_full_foil")) -> ()
      }
    }
    n6153 = Or(x="Parameters_set", y="Parameters_auto_set") -> (x .or. y?=w8960:bool)
    n6154 = case shown="True" w8960 {
      frame #0 {
      }
      frame #1 {
        n6155 = local read "Roll_side_select"() -> (w9089:enum32{"Left to Right", "Right to Left"})
        n6156 = case shown="\"Left to Right\", Default" w9089 {
          frame #0 {
            n6157 = stacked-sequence {
              frame #0 {
                n6158 = Wait (ms)(milliseconds to wait=u32 10) -> ()  [unwired: 1 out]
              }
              frame #1 {
                n6159 = local write "TC1_close_loop_coefficient"(sgl 100.0 ("TC2_close_loop_coefficient")) -> ()
              }
              frame #2 {
                n6160 = Wait (ms)(milliseconds to wait=u32 100) -> ()  [unwired: 1 out]
              }
              frame #3 {
                n6161 = local write "TC1_close_loop_set"(TRUE ("TC2_close_loop_set")) -> ()
              }
              frame #4 {
                n6162 = Wait (ms)(milliseconds to wait=u32 500) -> ()  [unwired: 1 out]
              }
              frame #5 {
                n6163 = local write "TC1_speed_gain_value"(sgl 0.0 ("TC2_speed_gain_value")) -> ()
              }
              frame #6 {
                n6164 = Wait (ms)(milliseconds to wait=u32 100) -> ()  [unwired: 1 out]
              }
              frame #7 {
                n6165 = local write "TC1_speed_gain_set"(TRUE ("TC2_speed_gain_set")) -> ()